vi "UHR-Fleezers Control (host) - 10.8MV_trial1.vi"() -> ()   [LabVIEW 2010] (continued)
            n273 = Concatenate Strings("1TJ3;\n2TJ3;\n3TJ3" ("Substring"), "\r") -> (w933:string)
            n274 = VISA Write(VISA resource name=w936, write buffer=w933) -> ()  [unwired: 1 in, 3 out]
          }
        }
      }
    }
  }
  n275 = disable-structure shown="Disabled" {
    disable-tunnel: w24 -> [w965 _]
    frame Disabled {
      w960 = T17 0 items=["Grayscale (U8)", "Grayscale (I16)", "Grayscale (SGL)", "Complex (CSG)", "RGB (U32)", "HSL (U32)", "RGB (U64)", "Grayscale (U16)"] ("Image Type")
      n276 = call <vilib>:"IMAQ Init.vi"("Interface Name"="img0") -> ("error out"=w962:errorcluster, "IMAQ Session Out"=w964:refnum<k11>)  [unwired: 9 in]
      n277 = call <vilib>:"IMAQ Grab Setup.vi"("error in (no error)"=w962, "IMAQ Session In"=w964) -> ("error out"=w958:errorcluster, "IMAQ Session Out"=w959:refnum<k11>)  [unwired: 8 in]
      n278 = call "IMAQ Create"("Image Name"="untitled", "Image Type"=w960) -> ("New Image"=w957:T2)  [unwired: 3 in, 1 out]
      n279 = call <vilib>:"Application Directory.vi"() -> ("Application Directory"=w944:path)
      n280 = Build Path(base path=w944, name or relative path="_trap_screen_positions") -> (appended path=w952:path)
      n281 = Open/Create/Replace File(file path (use dialog)=w952, operation (0:open)=T25."open or create", access (0:read/write)=enum16{"read/write", "read-only", "write-only"}."read/write") -> (refnum out=w954:refnum<file>)  [unwired: 3 in, 2 out]
      n282 = local read "Trap Sets"() -> (w946:u32)
      n283 = for "Load trap positions on video screen from file." {
        N: w946 -> [_]
        tunnel: [w972] -> w947
        tunnel: w954 -> [w971]
        tunnel: [w968] -> w943 mode=indexing
        w970 = 4
        n284 = for {
          N: w970 -> [_]
          tunnel: [w976] -> w972
          tunnel: w971 -> [w975]
          tunnel: w970 -> [w974]
          tunnel: [w973] -> w969 mode=indexing
          n285 = Read from Binary File(5:w974, 11:w975) -> (2:w973:i32, 3:w976:refnum<file>)  [unwired: 4 in, 2 out]
        }
        n286 = Array To Cluster(array=w969) -> (cluster=w968:T29)
      }
      n287 = node-c288() -> (w967:T26)  [unwired: 4 in]
      n288 = timed-loop "acquire video and stage position" {
        timing: w967 -> [_]
        timing-out: [_] -> w966
        tunnel: w959 -> [w995]
        tunnel: w958 -> [w994]
        tunnel: w957 -> [w993]
        tunnel: [w992] -> w939
        tunnel: [w989] -> w940
        tunnel: [w990] -> w938
        tunnel: w965 -> [_]
        shift-right: [w986] -> w956
        shift-left: w943 -> [w987]
        tunnel: w946 -> [w984]
        stop <- w991 stop-if-true
        n289 = node-c288() -> ()  [unwired: 1 in, 1 out]
        n290 = event shown="[2] \"Primary Video Display\": Mouse Down" {
          selector: _ -> [_ _ _ _]
          dyn-events: _ -> [_ _ _ _]
          timeout: 10 -> [_ _ _ _]
          tunnel: w995 -> [w1006 w1021 w1030 w1049]
          tunnel: w994 -> [w1005 w1023 w1028 w1051]
          tunnel: w993 -> [w1004 w1022 w1029 w1050]
          tunnel: [w1003 w1021 w1030 w1049] -> w992
          tunnel: [w996 w1025 FALSE FALSE] -> w991
          tunnel: [w1000 w1023 w1028 w1051] -> w990
          tunnel: [w999 w1022 w1029 w1050] -> w989
          tunnel: "radius" -> [_ _ w1035 _]
          tunnel: w987 -> [w997 w1024 w1033 _]
          tunnel: [w997 w1024 w1034 cluster{i32, i32, i32, i32}[] []] -> w986
          tunnel: w984 -> [_ _ w1026 _]
          event Timeout {
            n291 = event-data() -> ()  [unwired: 1 in, 2 out]
            n292 = call <vilib>:"IMAQ Grab Acquire.vi"("error in (no error)"=w1005, "Image In"=w1004, "IMAQ Session In"=w1006) -> ("error out"=w1001:errorcluster, "Image Out"=w1002:T2, "IMAQ Session Out"=w1003:refnum<k11>)  [unwired: 5 in, 1 out]
            n293 = case shown="True" "trap\nmarkers?" {
              tunnel: w997 -> [_ w1014]
              tunnel: w1002 -> [w1008 w1013]
              tunnel: w1001 -> [w1007 w1012]
              tunnel: [w1007 w1011] -> w1000
              tunnel: [w1008 w1009] -> w999
              frame False {
              }
              frame True {
                n294 = for {
                  tunnel: w1014 -> [w1020] mode=indexing
                  shift-right: [w1018] -> w1009
                  shift-left: w1013 -> [w1019]
                  tunnel: w1012 -> [w1017]
                  tunnel: [w1016] -> w1011
                  tunnel: u32 16711680 ("Color") -> [w1015]
                  n295 = call "IMAQ Overlay Oval"("Color"=w1015, "error in (no error)"=w1017, "Bounding Rectangle"=w1020, "Image"=w1019) -> ("error out"=w1016:errorcluster, "Image Out"=w1018:T2)  [unwired: 6 in]
                }
              }
            }
            "Primary Video Display" <- w999
            n296 = Unbundle By Name(w1001) -> ("status"=w996:bool)
          }
          event "Stop All": Value Change {
            n297 = event-data() -> ()  [unwired: 1 in, 5 out]
            n298 = local read "Stop All"() -> (w1025:bool)
          }
          event "Primary Video Display": Mouse Down {
            n299 = event-data() -> ()  [unwired: 1 in, 7 out]
            n300 = Array Size(array=w1033) -> (size(s)=w1032:i32)
            n301 = Less?(x=w1032, y=w1026) -> (x < y?=w1031:bool)
            n302 = case shown="True" w1031 {
              tunnel: w1035 -> [_ w1045]
              tunnel: w1033 -> [w1036 w1039]
              tunnel: [w1036 w1038] -> w1034
              frame False {
              }
              frame True {
                n303 = property on="Primary Video Display" class="ImageControl"() -> ("Last Mouse Position"=w1037:cluster{"X":i32, "Y":i32})  [unwired: 2 in, 2 out]
                n304 = Unbundle By Name(w1037) -> ("X"=w1047:i32, "Y"=w1046:i32)
                n305 = Add(x=w1046, y=w1045) -> (x+y=w1043:i32)
                n306 = Subtract(x=w1046, y=w1045) -> (x-y=w1041:i32)
                n307 = Add(x=w1047, y=w1045) -> (x+y=w1042:i32)
                n308 = Subtract(x=w1047, y=w1045) -> (x-y=w1044:i32)
                n309 = Bundle(w1044, w1043, w1042, w1041) -> (w1040:cluster{i32, i32, i32, i32})  [unwired: 1 in]
                n310 = Build Array (concatenate)(w1039, w1040) -> (w1038:T30)
              }
            }
          }
          event "clear markers": Value Change {
            n311 = event-data() -> ()  [unwired: 1 in, 5 out]
          }
        }
        n312 = node-c288() -> ()  [unwired: 1 in, 1 out]
      }
      n313 = node-c288(w966) -> ()  [unwired: 1 out]
      n314 = Set File Position(offset (in bytes) (0)=i64 0, refnum=w947, from (0:start)=enum16{"start", "end", "current"}."start") -> (refnum out=w948:refnum<file>)  [unwired: 1 in, 1 out]
      n315 = for "Write trap positions to file so they can be remembered\nwhen program is removed from memory" {
        tunnel: w956 -> [w980] mode=indexing
        tunnel: [w978] -> w955
        tunnel: w948 -> [w977]
        n316 = Cluster To Array(cluster=w980) -> (array=w979:i32[])
        n317 = for {
          tunnel: w979 -> [w983] mode=indexing
          tunnel: [w982] -> w978
          tunnel: w977 -> [w981]
          n318 = Write to Binary File(file (use dialog)=w981, data=w983) -> (refnum out=w982:refnum<file>)  [unwired: 4 in, 2 out]
        }
      }
      n319 = Close File(refnum=w955) -> ()  [unwired: 1 in, 2 out]
      n320 = call "IMAQ Dispose"("Image"=w940, "error in (no error)"=w938) -> ("error out"=w937:errorcluster)  [unwired: 4 in]
      n321 = call <vilib>:"IMAQ Stop.vi"("error in (no error)"=w937, "IMAQ Session In"=w939) -> ("error out"=w941:errorcluster, "IMAQ Session Out"=w942:refnum<k11>)  [unwired: 8 in]
      n322 = call <vilib>:"IMAQ Close.vi"("error in (no error)"=w941, "IMAQ Session In"=w942) -> ()  [unwired: 9 in, 1 out]
    }
    frame Enabled {
    }
  }
  n323 = node-c288(2 ("Processor")) -> (w15:T26)  [unwired: 3 in]
  n324 = node-c288() -> (w69:T26)  [unwired: 4 in]
  n325 = disable-structure shown="Enabled" {
    disable-tunnel: [w1058 _] -> w35
    disable-tunnel: w24 -> [w1057 _]
    frame Enabled {
      n326 = node-c288() -> (w1060:T26)  [unwired: 4 out]
      n327 = timed-loop "Rough control of MCL mirror stage (debugging)" {
        tunnel: w1057 -> [w1063]
        tunnel: [w1062] -> w1058
        timing: w1060 -> [_]
        timing-out: [_] -> w1059
        stop <- w1062 stop-if-true
        n328 = node-c288() -> ()  [unwired: 2 out]
        n329 = case shown="1" "MCL Mode" {
          tunnel: w1063 -> [_ w1066 w1170]
          frame 0, Default {
            # "manual positioning"
          }
          frame 1 {
            # "sinusoidal wave"
            n330 = node-c288() -> (w1068:T26)  [unwired: 4 out]
            n331 = timed-loop "Oscillate MCL mirror" {
              timing: w1068 -> [_]
              timing-out: [_] -> w1067
              tunnel: w1066 -> [w1107]
              i -> [w1106]
              stop <- w1069 stop-if-true
              n332 = node-c288() -> (w1105:i64)  [unwired: 1 out]
              n333 = Multiply(x="AO1", y=32767.0) -> (x*y=w1101:dbl)
              n334 = Multiply(x="AO2", y=32767.0) -> (x*y=w1096:dbl)
              n335 = Divide(x=w1101, y=10.0) -> (x/y=w1102:dbl)
              n336 = Divide(x=w1096, y=10.0) -> (x/y=w1097:dbl)
              n337 = To Word Integer(number=w1102) -> (16bit integer=w1094:i16)
              n338 = To Word Integer(number=w1097) -> (16bit integer=w1093:i16)
              n339 = Divide(x=w1105, y=i64 1000) -> (x/y=w1076:dbl)
              n340 = Multiply(x=w1076, y=w1106) -> (x*y=w1087:dbl)
              n341 = Multiply(x="Osc. freq. (Hz) 2", y=6.283185307179586) -> (x*y=w1088:dbl)
              n342 = Multiply(x=w1088, y=w1087) -> (x*y=w1086:dbl)
              n343 = Sine(x=w1086) -> (sin(x)=w1085:dbl)
              n344 = Multiply(x=w1085, y="Osc. amp. (V)") -> (x*y=w1083:dbl)
              n345 = Add(x=w1083, y="Osc. center (V)") -> (x+y=w1081:dbl)
              n346 = Divide(x=w1081, y=10.0) -> (x/y=w1079:dbl)
              n347 = Multiply(x=w1079, y=32767.0) -> (x*y=w1074:dbl)
              n348 = Select(t=w1074, s="Scan axis", f=w1094) -> (s? t:f=w1092:dbl)
              n349 = Select(t=w1093, s="Scan axis", f=w1074) -> (s? t:f=w1091:dbl)
              n350 = local read "MCL Mode"() -> (w1073:u16)
              n351 = Not Equal?(x=w1073, y=u16 1) -> (x != y?=w1070:bool)
              n352 = local read "Stop All"() -> (w1071:bool)
              n353 = xnode "Read/Write Control"("FPGA VI Reference In"=w1107, "AO1"=w1092, "AO2"=w1091) -> ()  [unwired: 1 in, 2 out]
              n354 = Compound Arithmetic op=OR(w1071, w1070) -> (w1069:bool)
              n355 = node-c288() -> ()  [unwired: 2 out]
            }
            n356 = node-c288(w1067) -> ()  [unwired: 1 out]
          }
          frame 2 {
            # "linear scan"
            n357 = case shown="True" "Start Scan" {
              tunnel: w1170 -> [_ w1182]
              frame False {
              }
              frame True {
                n358 = Subtract(x="End (V)", y="Begin (V)") -> (x-y=w1178:dbl)
                n359 = Decrement(x="N Points") -> (x-1=w1177:dbl)
                n360 = Divide(x=w1178, y=w1177) -> (x/y=w1175:dbl)
                n361 = for {
                  N: "N Points" -> [_]
                  tunnel: "Begin (V)" -> [w1195]
                  tunnel: w1182 -> [w1187]
                  tunnel: [w1186] -> w1181 mode=indexing
                  tunnel: w1175 -> [w1185]
                  tunnel: [w1183] -> w1174 mode=indexing
                  i -> [w1194]
                  n362 = Multiply(x=w1185, y=w1194) -> (x*y=w1193:dbl)
                  n363 = Add(x=w1195, y=w1193) -> (x+y=w1190:dbl)
                  n364 = local read "Scan axis"() -> (w1184:bool)
                  n365 = local read "AO1"() -> (w1192:dbl)
                  n366 = local read "AO2"() -> (w1191:dbl)
                  n367 = Select(t=w1190, s=w1184, f=w1192) -> (s? t:f=w1189:dbl)
                  n368 = Select(t=w1191, s=w1184, f=w1190) -> (s? t:f=w1188:dbl)
                  n369 = flat-sequence {
                    tunnel: w1189 -> [w1199]
                    tunnel: w1188 -> [w1198]
                    tunnel: w1187 -> [w1196]
                    tunnel: [w1266] -> w1186
                    tunnel: [w1265] -> w1183
                    frame #0 {
                      w1202 = 10.0 ("y")
                      w1197 = 32767.0 ("y")
                      n370 = Multiply(x=w1199, y=w1197) -> (x*y=w1205:dbl)
                      n371 = Multiply(x=w1198, y=w1197) -> (x*y=w1203:dbl)
                      n372 = Divide(x=w1205, y=w1202) -> (x/y=w1206:dbl)
                      n373 = Divide(x=w1203, y=w1202) -> (x/y=w1204:dbl)
                      n374 = To Word Integer(number=w1206) -> (16bit integer=w1200:i16)
                      n375 = To Word Integer(number=w1204) -> (16bit integer=w1201:i16)
                      n376 = xnode "Read/Write Control"("FPGA VI Reference In"=w1196, "AO1"=w1200, "AO2"=w1201) -> ()  [unwired: 1 in, 2 out]
                    }
                    frame #1 {
                      n377 = Wait (ms)(milliseconds to wait="DAQ Delay (ms)") -> ()  [unwired: 1 out]
                    }
                    frame #2 {
                      n378 = local read "Slow mean"() -> (w1266:dbl)
                      n379 = local read "Sigma"() -> (w1265:dbl)
                    }
                  }
                }
                n380 = Bundle("Begin (V)"="Begin (V)", w1175, w1181) -> (→"MCL Scan":cluster{"Begin (V)":dbl, dbl, dbl[]})  [unwired: 1 out]
                n381 = Bundle("Begin (V)"="Begin (V)", w1175, w1174) -> (→"MCL Scan 2":cluster{"Begin (V)":dbl, dbl, dbl[]})  [unwired: 1 out]
              }
            }
          }
        }
        n382 = local read "Stop All"() -> (w1062:bool)
        n383 = node-c288() -> ()  [unwired: 2 out]
      }
      n384 = node-c288(w1059) -> ()  [unwired: 1 out]
    }
    frame Disabled {
    }
  }
  n385 = timed-loop "Control parameters (event loop)" {
    tunnel: w24 -> [w1272]
    shift-right: [w1271] -> _
    shift-left: errorcluster {"status"=FALSE, "code"=0, "source"=""} ("error out") -> [w1270]
    tunnel: [w1269] -> w37
    timing: w15 -> [_]
    timing-out: [_] -> w14
    stop <- w1269 stop-if-true
    n386 = node-c288() -> ()  [unwired: 1 in, 1 out]
    n387 = event shown="[6] \"BD 1 Frequency 1 (MHz)\", \"BD 1 Frequency 2 (MHz)\", \"BD 1 Frequency 3 (MHz)\", \"BD 2 Frequency 1 (MHz)\", \"BD 2 Frequency 2 (MHz)\", \"BD 2 Frequency 3 (MHz)\", \"Trap Delta (MHz)\": Value Change" {
      selector: _ -> [_ _ _ _ _ _ _ _ _ _ _ _ _ _ _ _ _ _ _ _ _ _ _ _ _ _ _ _ _ _ _ _ _ _ _ _ _ _ _ _ _ _ _ _ _ _ _ _ _ _ _ _ _ _ _]
      dyn-events: _ -> [_ _ _ _ _ _ _ _ _ _ _ _ _ _ _ _ _ _ _ _ _ _ _ _ _ _ _ _ _ _ _ _ _ _ _ _ _ _ _ _ _ _ _ _ _ _ _ _ _ _ _ _ _ _ _]
      timeout: _ -> [_ _ _ _ _ _ _ _ _ _ _ _ _ _ _ _ _ _ _ _ _ _ _ _ _ _ _ _ _ _ _ _ _ _ _ _ _ _ _ _ _ _ _ _ _ _ _ _ _ _ _ _ _ _ _]
      tunnel: w1272 -> [w1310 _ _ _ w1432 _ w1529 _ w1593 _ _ _ w1788 _ _ w1890 w2034 w2098 w2173 w2327 w2404 w2535 w2631 w2717 w2803 w2889 w2975 w3061 w3154 w3318 w3529 _ w3674 w3811 _ w4018 w4060 w4108 w4187 w4229 _ w4275 _ _ _ _ w4466 _ w4559 w4600 w4647 w4835 w4884 _ w4946]
      tunnel: [w1309 _ _ _ w1422 _ w1528 _ w1556 _ w1753 _ w1767 _ _ w1889 w2030 w2095 w2170 w2326 w2402 w2534 w2625 w2711 w2797 w2883 w2969 w3055 w3152 w3317 w3527 _ w3672 w3809 _ w4016 w4058 w4098 w4185 w4227 _ w4273 _ _ _ _ w4464 _ _ _ _ _ _ _ _] -> w1271
      tunnel: w1270 -> [w1308 _ _ _ w1431 _ w1527 _ w1588 _ w1753 _ w1787 _ _ w1888 w2029 w2094 w2169 w2325 w2403 w2533 w2630 w2716 w2802 w2888 w2974 w3060 w3153 w3316 w3528 _ w3673 w3810 _ w4017 w4059 w4107 w4186 w4228 _ w4274 _ _ _ _ w4465 _ w4558 w4599 w4646 w4834 w4883 _ w4945]
      tunnel: [_ _ _ _ _ _ _ _ _ _ w1752 _ _ _ _ _ _ _ _ _ _ _ _ _ _ _ _ _ _ _ _ _ _ _ _ _ _ _ _ _ _ _ _ _ _ _ _ _ _ _ _ _ _ _ _] -> w1269
      tunnel: [_ _ _ _ _ _ _ "Round T1 X" _ _ _ _ _ _ _ _ _ _ _ _ _ _ _ _ _ _ _ _ _ _ _ _ _ _ _ _ _ _ _ _ _ _ _ _ _ _ _ _ _ _ _ _ _ _ _] -> _
      tunnel: [_ _ _ "Adjust Scale\nto Mean" _ _ _ _ _ _ _ _ _ _ _ _ _ _ _ _ _ _ _ _ _ _ _ _ _ _ _ _ _ _ _ _ _ _ _ _ _ _ _ _ _ _ _ _ _ _ _ _ "Set SP to Reading" _ _] -> _
      tunnel: [_ _ _ _ _ _ _ _ _ "Round T2 X" _ "Delayed Interlace Start" _ _ _ _ _ _ _ _ _ _ _ _ _ _ _ _ _ _ _ _ _ _ _ _ _ _ _ _ _ _ _ _ _ _ _ _ _ _ _ _ _ _ _] -> _
      event "AI Count (ticks)", "Sets to FIFO (Traps)", "Save ave N", "FPGA Ave.", "# Samples/channel", "N sets to save": Value Change {
        # "So that if 'Save ave N' is updated, the AOD scanning code updates too."
        n388 = event-data() -> ()  [unwired: 6 out]
        n389 = local read "AI Count (ticks)"() -> (w1290:u32)
        n390 = Boolean To (0,1)(Boolean="Sets to FIFO (Traps)") -> (0, 1=w1300:cluster{"Set 1":i16, "Set 2":i16, "Set 3":i16})
        n391 = xnode "Read/Write Control"("FPGA VI Reference In"=w1310, "error in"=w1308, "ai count"=w1290, "AI1 Sets to FIFO"="Sets to FIFO (Traps)", "N of AI1 Int Acq Sets"="N Acq Sets (Traps + Fl.)") -> ("error out"=w1309:errorcluster)  [unwired: 1 out]
        n392 = Cluster To Array(cluster=w1300) -> (array=w1299:i16[])
        n393 = To Unsigned Long Integer(number=w1299) -> (unsigned 32bit integer=w1279:u32[])
        n394 = local read "Scan steps (AOD)"() -> (w1301:u64)
        n395 = Multiply(x=w1290, y="N Acq Sets (Traps + Fl.)") -> (x*y=w1288:u32)
        n396 = Divide(x=40000000.0, y=w1290) -> (x/y=w1282:dbl)
        "AI rate (Hz)" <- w1282
        "Ave. Rate (Hz)" <- w1282
        n397 = Add Array Elements(numeric array=w1279) -> (sum=w1291:u32)
        "Trap Sets" <- w1291
        n398 = Reciprocal(x=w1282) -> (1/x=→"Ave. Period (s)":dbl)
        n399 = property on="Scan steps (AOD)" class="DigNum (strict)"("Val(Sgnl)"=w1301) -> ()  [unwired: 2 in, 2 out]
        n400 = Divide(x=w1282, y="N Acq Sets (Traps + Fl.)") -> (x/y=w1305:dbl)
        "Data Rate (Hz)" <- w1305
        n401 = Reciprocal(x=w1305) -> (1/x=→"Data Period (s)":dbl)
        n402 = local read "Save ave N"() -> (w1304:dbl)
        n403 = Divide(x=w1305, y=w1304) -> (x/y=w1303:dbl)
        "Save Data Rate (Hz)" <- w1303
        n404 = Reciprocal(x=w1303) -> (1/x=→"Save Data Period (s)":dbl)
        n405 = Multiply(x=w1288, y="# Samples/trap") -> (x*y=w1286:u32)
        "Counts/DMA" <- w1286
        n406 = property on="Trap Disp. Downsample" class="DigNum (strict)"("Maximum"="# Samples/trap") -> ()  [unwired: 2 in, 2 out]
        n407 = Multiply(x=w1291, y="# Samples/trap") -> (x*y=w1280:u32)
        "# Samples/channel" <- w1280
        n408 = Multiply(x=w1280, y=u32 8) -> (x*y=→"Trap AI Elements/DMA read":u32)
        n409 = local read "APD Int. Count"() -> (w1287:u32)
        n410 = Multiply(x=w1280, y=u32 3) -> (x*y=→"Trap Pos Elements/DMA read":u32)
        n411 = Divide(x=w1286, y=w1287) -> (x/y=w1277:dbl)
        "APD Samples/FIFO Acq." <- w1277
        n412 = Divide(x=w1286, y=40000000.0) -> (x/y=w1284:dbl)
        "DMA Update Period (s)" <- w1284
        n413 = Multiply(x=2.0, y=w1277) -> (x*y=→"APD Elements/DMA read":dbl)
        n414 = property on="APD Disp. Downsample" class="DigNum (strict)"("Maximum"=w1277) -> ()  [unwired: 2 in, 2 out]
        n415 = local read "N sets to save"() -> (w1297:u32)
        n416 = Multiply(x=w1284, y=w1297) -> (x*y=→"Total Time (s)":dbl)
        "FPGA Averaging" <- FALSE ("FPGA Averaging")
      }
      event "Rescale on Mean": Value Change {
        n417 = event-data() -> ()  [unwired: 7 out]
        n418 = And(x=FALSE, y="Rescale on Mean") -> (x .and. y?=w1397:bool)
        n419 = local write "Rescale on Mean"(w1397) -> ()
        n420 = local read "Bead Mean (nm)"() -> (w1402:dbl)
        n421 = Add(x="Amplitude (nm)", y=w1402) -> (x+y=w1400:dbl)
        n422 = Subtract(x=w1402, y="Amplitude (nm)") -> (x-y=w1399:dbl)
        n423 = property on="Bead Separation" class="WFChart (strict)"("YScale.Minimum"=w1399) -> ()  [unwired: 2 in, 2 out]
        n424 = property on="Bead Separation" class="WFChart (strict)"("YScale.Maximum"=w1400) -> ()  [unwired: 2 in, 2 out]
      }
      event "Detector Type": Value Change {
        n425 = event-data() -> ()  [unwired: 7 out]
        n426 = local read "AI labels"() -> (w1403:string[])
        n427 = property on="High Res. Display" class="Ring (strict)"("Strings []"=w1403) -> ()  [unwired: 2 in, 2 out]
        n428 = Build Array (concatenate)(w1403, "none") -> (w1404:string[])
        n429 = property on="FFT 1 Choice 1" class="Ring (strict)"("Strings []"=w1404) -> ()  [unwired: 2 in, 2 out]
        n430 = property on="FFT 1 Choice 2" class="Ring (strict)"("Strings []"=w1404) -> ()  [unwired: 2 in, 2 out]
        n431 = property on="FFT 2 Choice 1" class="Ring (strict)"("Strings []"=w1404) -> ()  [unwired: 2 in, 2 out]
        n432 = property on="FFT 2 Choice 2" class="Ring (strict)"("Strings []"=w1404) -> ()  [unwired: 2 in, 2 out]
        n433 = Bundle("APD 1", "APD 2") -> (w1407:cluster{string, string})  [unwired: 1 out]
        n434 = Cluster To Array(cluster=w1407) -> (array=w1405:string[])
        n435 = Build Array (concatenate)(w1405, w1404) -> (w1409:string[])
        n436 = Array Size(array=w1409) -> (size(s)=w1410:i32)
        n437 = property on="Signals to Plot" class="LstBox (strict)"("Item Names"=w1409) -> ()  [unwired: 2 in, 2 out]
        n438 = property on="Signals to Plot" class="LstBox (strict)"("Number of Rows"=w1410) -> ()  [unwired: 2 in, 2 out]
        n439 = property on="All Signals" class="WFChart (strict)"("LegNumRows"=w1410) -> ()  [unwired: 2 in, 2 out]
      }
      event "Adjust Scale\nto Mean": Value Change {
        n440 = event-data() -> ()  [unwired: 7 out]
        n441 = local read "APD 1 Rate (Hz)"() -> (w1419:dbl)
        n442 = Multiply(x=1000.0, y="Above (kHz)") -> (x*y=w1417:dbl)
        n443 = Multiply(x=1000.0, y="Below (kHz)") -> (x*y=w1415:dbl)
        n444 = Add(x=w1417, y=w1419) -> (x+y=w1412:dbl)
        n445 = Subtract(x=w1419, y=w1415) -> (x-y=w1413:dbl)
        n446 = property on="APD Chart" class="WFChart (strict)"("YScale.Minimum"=w1413) -> ()  [unwired: 2 in, 2 out]
        n447 = property on="APD Chart" class="WFChart (strict)"("YScale.Maximum"=w1412) -> ()  [unwired: 2 in, 2 out]
      }
      event "Phase adj. (AI1)", "+ phase (AI1)", "- phase (AI1)": Value Change {
        n448 = event-data() -> ()  [unwired: 7 out]
        n449 = Negate(x="Phase adj. (AI1)") -> (-x=w1429:i16)
        n450 = Select(t=w1429, s="- phase (AI1)", f="Phase adj. (AI1)") -> (s? t:f=w1428:i16)
        n451 = xnode "Read/Write Control"("FPGA VI Reference In"=w1432, "error in"=w1431, "Phase count adjustment"=w1428) -> ("FPGA VI Reference Out"=w1427:T19, "error out"=w1426:errorcluster)
        n452 = Or(x="- phase (AI1)", y="+ phase (AI1)") -> (x .or. y?=w1423:bool)
        n453 = xnode "Read/Write Control"("FPGA VI Reference In"=w1427, "error in"=w1426, "+ phase"=w1423) -> ("error out"=w1422:errorcluster)  [unwired: 1 out]
      }
      event "Signals to Plot": Double Click {
        w1510 = u32 9868950 ("Color Box")
        n454 = event-data() -> ("Row"=w1512:i32)  [unwired: 9 out]
        n455 = property on="All Signals" class="WFChart (strict)"("Active Plot"=w1512) -> (error out=w1523:errorcluster)  [unwired: 2 in, 1 out]
        n456 = property on="All Signals" class="WFChart (strict)" props=["Plot", "Visible?", "Plot", "Plot Color"](error in=w1523) -> (error out=w1522:errorcluster, "Plot.Visible?"=w1521:bool)  [unwired: 1 in, 2 out]
        n457 = Select(t=FALSE ("Plot.Visible"), s=w1521, f=TRUE ("Plot.Visible")) -> (s? t:f=w1516:bool)
        n458 = property on="All Signals" class="WFChart (strict)"(error in=w1522, "Plot.Visible?"=w1516) -> (error out=w1518:errorcluster)  [unwired: 1 in, 1 out]
        n459 = property on="All Signals" class="WFChart (strict)"(error in=w1518) -> (error out=w1513:errorcluster, "Plot.Plot Color"=w1517:u32)  [unwired: 1 in, 1 out]
        n460 = property on="Signals to Plot" class="LstBox (strict)"(error in=w1513, "Active Row"=w1512) -> (error out=w1511:errorcluster)  [unwired: 1 in, 1 out]
        n461 = Select(t=w1517, s=w1516, f=u32 0) -> (s? t:f=w1514:u32)
        n462 = property on="Signals to Plot" class="LstBox (strict)"(error in=w1511, "CellFontColor"=w1514, "SelColor"=w1510, "CellBG"=w1510, "CellFontSize"=u32 20 ("Active Row:Cell Font:Size"), "CellFontBold"=TRUE ("Active Row:Cell Font:Bold")) -> ()  [unwired: 1 in, 2 out]
      }
      event "BD 1 Frequency 1 (MHz)", "BD 1 Frequency 2 (MHz)", "BD 1 Frequency 3 (MHz)", "BD 2 Frequency 1 (MHz)", "BD 2 Frequency 2 (MHz)", "BD 2 Frequency 3 (MHz)", "Trap Delta (MHz)": Value Change {
        # "anytime one of the frequencies is changed, write it to the RF board UNLESS Set 2 is being oscillated. The oscillation\nscript writes the frequencies to the RF board."
        n463 = event-data() -> ("CtlRef"=w1526:refnum<vi>)  [unwired: 6 out]
        n464 = control-ref of="Trap Delta (MHz)"() -> (w1525:refnum<vi>)
        n465 = Equal?(x=w1525, y=w1526) -> (x = y?=w1524:bool)
        n466 = case shown="False" "Oscillate Set 2" {
          tunnel: w1529 -> [w1549 _]
          tunnel: [w1548 w1552] -> w1528
          tunnel: w1527 -> [w1547 w1552]
          tunnel: w1524 -> [w1533 _]
          frame False {
            n467 = local read "BD 1 Frequency 1 (MHz)"() -> (w1531:dbl)
            n468 = local read "BD 1 Frequency 2 (MHz)"() -> (w1535:dbl)
            n469 = Add(x=w1531, y="Trap Delta (MHz)") -> (x+y=w1534:dbl)
            n470 = Select(t=w1534, s=w1533, f=w1535) -> (s? t:f=w1532:dbl)
            n471 = local read "Y RF Frequency Limits (MHz)"() -> (w1537:T16)
            n472 = local read "X RF Frequency Limits (MHz)"() -> (w1538:T16)
            n473 = local read "BD 1 Frequency 3 (MHz)"() -> (w1550:dbl)
            n474 = local write "BD 1 Frequency 2 (MHz)"(w1532) -> ()
            n475 = local read "BD 2 Frequency 1 (MHz)"() -> (w1541:dbl)
            n476 = local read "BD 2 Frequency 2 (MHz)"() -> (w1540:dbl)
            n477 = local read "BD 2 Frequency 3 (MHz)"() -> (w1551:dbl)
            n478 = call "set RF board frequency - interlace.vi"("Board 2 Frequency Limits"=w1537, "Board 1 Frequency Limits"=w1538, "error in"=w1547, "FPGA VI Reference In"=w1549, "Board 2 Frequency 3 (MHz)"=w1551, "Board 1 Frequency 3 (MHz)"=w1550, "Board 2 Frequency 2 (MHz)"=w1540, "Board 2 Frequency 1 (MHz)"=w1541, "Board 1 Frequency 2 (MHz)"=w1532, "Board 1 Frequency 1  (MHz)"=w1531) -> ("error out"=w1548:errorcluster)  [unwired: 1 out]
            n479 = Subtract(x=w1541, y=w1540) -> (x-y=w1545:dbl)
            n480 = Subtract(x=w1532, y=w1531) -> (x-y=w1546:dbl)
            n481 = Square(x=w1545) -> (x^2=w1543:dbl)
            n482 = Square(x=w1546) -> (x^2=w1544:dbl)
            n483 = Add(x=w1544, y=w1543) -> (x+y=w1542:dbl)
            n484 = Square Root(x=w1542) -> (sqrt(x)=w1539:dbl)
            n485 = local write "Trap Delta (MHz)"(w1539) -> ()
            n486 = property on="Initial delta (MHz)" class="DigNum (strict)"("Val(Sgnl)"=w1539) -> ()  [unwired: 2 in, 2 out]
          }
          frame True {
          }
        }
      }
      event "Round T1 X": Value Change {
        n487 = event-data() -> ()  [unwired: 7 out]
        n488 = local read "BD 1 Frequency 1 (MHz)"() -> (w1555:dbl)
        n489 = Round To Nearest(number=w1555) -> (nearest integer value=w1554:dbl)
        n490 = property on="BD 1 Frequency 1 (MHz)" class="DigNum (strict)"("Val(Sgnl)"=w1554) -> ()  [unwired: 2 in, 2 out]
      }
      event "Restart RF": Value Change {
        n491 = event-data() -> ()  [unwired: 7 out]
        n492 = xnode "Read/Write Control"("FPGA VI Reference In"=w1593, "error in"=w1588, "FPGA Controls  RF Box"=FALSE) -> ("FPGA VI Reference Out"=w1592:T19, "error out"=w1587:errorcluster)
        n493 = local read "Y RF Amplitude Limits (%)"() -> (w1568:T16)
        n494 = local read "X RF Amplitude Limits (%)"() -> (w1569:T16)
        n495 = local read "X RF Frequency Limits (MHz)"() -> (w1571:T16)
        n496 = local read "Y RF Frequency Limits (MHz)"() -> (w1570:T16)
        n497 = xnode "Read/Write Control"("FPGA VI Reference In"=w1592, "error in"=w1587, "Direct RF Box  Communication"=TRUE) -> ("FPGA VI Reference Out"=w1591:T19, "error out"=w1586:errorcluster)
        n498 = local read "BD 2 Frequency 3 (MHz)"() -> (w1578:dbl)
        n499 = local read "BD 2 Frequency 2 (MHz)"() -> (w1579:dbl)
        n500 = local read "BD 1 Frequency 3 (MHz)"() -> (w1582:dbl)
        n501 = local read "BD 1 Frequency 1 (MHz)"() -> (w1583:dbl)
        n502 = local read "BD 2 Frequency 1 (MHz)"() -> (w1580:dbl)
        n503 = local read "BD 1 Frequency 2 (MHz)"() -> (w1581:dbl)
        n504 = call "Initialize RF boards - interlace 3.vi"("error in"=w1586, "FPGA VI Reference In"=w1591) -> ("error out"=w1585:errorcluster, "FPGA VI Reference Out"=w1590:T19)
        n505 = local read "BD 2 Amplitude 2 (%)"() -> (w1573:dbl)
        n506 = local read "BD 2 Amplitude 1 (%)"() -> (w1574:dbl)
        n507 = local read "BD 2 Amplitude 3 (%)"() -> (w1572:dbl)
        n508 = local read "BD 1 Amplitude 3 (%)"() -> (w1577:dbl)
        n509 = local read "BD 1 Amplitude 1 (%)"() -> (w1576:dbl)
        n510 = local read "BD 1 Amplitude 2 (%)"() -> (w1575:dbl)
        n511 = call "set RF board frequency - interlace.vi"("Board 2 Frequency Limits"=w1570, "Board 1 Frequency Limits"=w1571, "error in"=w1585, "FPGA VI Reference In"=w1590, "Board 2 Frequency 3 (MHz)"=w1578, "Board 1 Frequency 3 (MHz)"=w1582, "Board 2 Frequency 2 (MHz)"=w1579, "Board 2 Frequency 1 (MHz)"=w1580, "Board 1 Frequency 2 (MHz)"=w1581, "Board 1 Frequency 1  (MHz)"=w1583) -> ("error out"=w1584:errorcluster, "FPGA VI Reference Out"=w1589:T19)
        n512 = call "set RF board amplitude - interlace.vi"("Board 2 Amplitude Limits"=w1568, "Board 1 Amplitude Limits"=w1569, "error in"=w1584, "FPGA VI Reference In"=w1589, "Board 2 Amplitude 3 (%)"=w1572, "Board 1 Amplitude 3 (%)"=w1577, "Board 2 Amplitude 2 (%)"=w1573, "Board 2 Amplitude 1 (%)"=w1574, "Board 1 Amplitude 2 (%)"=w1575, "Board 1 Amplitude 1 (%)"=w1576) -> ("error out"=w1561:errorcluster, "FPGA VI Reference Out"=w1565:T19)
        n513 = xnode "Read/Write Control"("FPGA VI Reference In"=w1565, "error in"=w1561, "Direct RF Box  Communication"=FALSE) -> ("FPGA VI Reference Out"=w1564:T19, "error out"=w1563:errorcluster)
        n514 = flat-sequence {
          tunnel: w1563 -> [w1594]
          tunnel: [w1594] -> w1562
          frame #0 {
            n515 = Wait (ms)(milliseconds to wait=u32 50) -> ()  [unwired: 1 out]
          }
        }
        n516 = xnode "Read/Write Control"("FPGA VI Reference In"=w1564, "error in"=w1562, "FPGA Controls  RF Box"=TRUE) -> ("error out"=w1557:errorcluster)  [unwired: 1 out]
        n517 = property on="Restart RF" class="Bool (strict)"(error in=w1557, "Value"=FALSE ("Restart RF")) -> (error out=w1556:errorcluster)  [unwired: 1 in, 1 out]
      }
      event "Round T2 X": Value Change {
        n518 = event-data() -> ()  [unwired: 7 out]
        n519 = local read "BD 1 Frequency 2 (MHz)"() -> (w1749:dbl)
        n520 = Round To Nearest(number=w1749) -> (nearest integer value=w1748:dbl)
        n521 = property on="BD 1 Frequency 2 (MHz)" class="DigNum (strict)"("Val(Sgnl)"=w1748) -> ()  [unwired: 2 in, 2 out]
      }
      event "Stop All": Value Change {
        n522 = event-data() -> ()  [unwired: 7 out]
        n523 = call "hamilton_controller.vi"("action"=T22."DISCONNECT") -> ()  [unwired: 10 in, 1 out]
        n524 = local read "Stop All"() -> (w1752:bool)
      }
      event "Delayed Interlace Start": Value Change {
        n525 = event-data() -> ()  [unwired: 7 out]
        n526 = flat-sequence {
          frame #0 {
            n527 = Multiply(x="Delay to Interlace (s)", y=1000.0) -> (x*y=w1755:dbl)
            n528 = Wait (ms)(milliseconds to wait=w1755) -> ()  [unwired: 1 out]
          }
          frame #1 {
            n529 = property on="Green laser mode" class="RadioBtnsControl (strict)"("Val(Sgnl)"=enum32{"Laser ON", "Laser OFF", "Interlace"}."Interlace" ("Value (Signaling)")) -> ()  [unwired: 2 in, 2 out]
          }
        }
      }
      event "BD 1 Amplitude 1 (%)", "BD 1 Amplitude 2 (%)", "BD 1 Amplitude 3 (%)", "BD 2 Amplitude 1 (%)", "BD 2 Amplitude 2 (%)", "BD 2 Amplitude 3 (%)", "Trap 1 ON", "Trap 2 ON", "Trap 3 ON", "Feedback On/Off", "All FB On/Off": Value Change {
        w1779 = i16 1 ("f")
        n530 = event-data() -> ()  [unwired: 7 out]
        n531 = local write "Trap 1 (ON/OFF)"("Trap 1 ON") -> ()
        n532 = local write "Trap 2 (ON/OFF)"("Trap 2 ON") -> ()
        n533 = Boolean To (0,1)(Boolean="Trap 3 ON") -> (0, 1=w1780:i16)
        n534 = Boolean To (0,1)(Boolean="Trap 1 ON") -> (0, 1=w1781:i16)
        n535 = Boolean To (0,1)(Boolean="Trap 2 ON") -> (0, 1=w1782:i16)
        n536 = Select(t=w1782, s="Trap ON/OFF X or Y Amp?", f=w1779) -> (s? t:f=w1777:i16)
        n537 = Select(t=w1781, s="Trap ON/OFF X or Y Amp?", f=w1779) -> (s? t:f=w1778:i16)
        n538 = Select(t=w1780, s="Trap ON/OFF X or Y Amp?", f=w1779) -> (s? t:f=w1776:i16)
        n539 = Select(t=w1779, s="Trap ON/OFF X or Y Amp?", f=w1782) -> (s? t:f=w1774:i16)
        n540 = Select(t=w1779, s="Trap ON/OFF X or Y Amp?", f=w1781) -> (s? t:f=w1775:i16)
        n541 = Select(t=w1779, s="Trap ON/OFF X or Y Amp?", f=w1780) -> (s? t:f=w1773:i16)
        n542 = And(x="All FB On/Off", y="Feedback On/Off") -> (x .and. y?=w1771:cluster{"Set 1":bool, "Set 2":bool})
        n543 = local read "BD 1 Amplitude 1 (%)"() -> (w1791:dbl)
        n544 = local read "BD 1 Amplitude 2 (%)"() -> (w1790:dbl)
        n545 = local read "BD 1 Amplitude 3 (%)"() -> (w1789:dbl)
        n546 = Unbundle By Name(w1771) -> ("Set 1"=w1766:bool, "Set 2"=w1763:bool)
        n547 = local read "Y RF Amplitude Limits (%)"() -> (w1759:T16)
        n548 = local read "X RF Amplitude Limits (%)"() -> (w1760:T16)
        n549 = local read "BD 2 Amplitude 1 (%)"() -> (w1792:dbl)
        n550 = local read "BD 2 Amplitude 2 (%)"() -> (w1793:dbl)
        n551 = local read "BD 2 Amplitude 3 (%)"() -> (w1794:dbl)
        n552 = And(x="Trap 2 ON", y=w1763) -> (x .and. y?=w1761:bool)
        n553 = And(x="Trap 1 ON", y=w1766) -> (x .and. y?=w1764:bool)
        n554 = Multiply(x=w1778, y=w1791) -> (x*y=w1786:dbl)
        n555 = Multiply(x=w1790, y=w1777) -> (x*y=w1784:dbl)
        n556 = Multiply(x=w1789, y=w1776) -> (x*y=w1785:dbl)
        n557 = Multiply(x=w1792, y=w1775) -> (x*y=w1795:dbl)
        n558 = Multiply(x=w1793, y=w1774) -> (x*y=w1796:dbl)
        n559 = Multiply(x=w1794, y=w1773) -> (x*y=w1797:dbl)
        n560 = call "set RF board amplitude - interlace.vi"("Board 2 Amplitude Limits"=w1759, "Board 1 Amplitude Limits"=w1760, "error in"=w1787, "FPGA VI Reference In"=w1788, "Board 2 Amplitude 3 (%)"=w1797, "Board 1 Amplitude 3 (%)"=w1785, "Board 2 Amplitude 2 (%)"=w1796, "Board 2 Amplitude 1 (%)"=w1795, "Board 1 Amplitude 2 (%)"=w1784, "Board 1 Amplitude 1 (%)"=w1786) -> ("error out"=w1768:errorcluster, "FPGA VI Reference Out"=w1769:T19)
        n561 = xnode "Read/Write Control"("FPGA VI Reference In"=w1769, "error in"=w1768, "FB On/Off Set 1"=w1764, "FB On/Off Set 2"=w1761) -> ("error out"=w1767:errorcluster)  [unwired: 1 out]
      }
      event "Load parameters": Value Change {
        n562 = event-data() -> ()  [unwired: 7 out]
        n563 = property on="Saved AOD Raster Scan Parameter Sets" class="Arr (strict)"() -> ("Index Values"=w1867:u32[])  [unwired: 2 in, 2 out]
        n564 = Index Array(array=w1867, index=0) -> (element=w1864:u32)
        n565 = local write "Load parameters"(FALSE ("Load parameters")) -> ()
        n566 = Index Array(array="Saved AOD Raster Scan Parameter Sets", index=w1864) -> (element=w1863:T32)
        n567 = Unbundle By Name(w1863) -> ("Scan Range AOD (nm) 2"=w1862:dbl, "Step Size AOD (nm) 2"=w1861:dbl, "Scan Speed AOD (nm/s) 2"=w1860:dbl, "Number of scans (AOD) 2"=w1859:u16)
        n568 = flat-sequence {
          tunnel: w1862 -> [w1870]
          tunnel: w1861 -> [w1869]
          tunnel: w1860 -> [w1868]
          tunnel: w1859 -> [w1871]
          frame #0 {
            n569 = local write "Scan Speed (nm/s)"(w1868) -> ()
            n570 = local write "Scan Range (nm)"(w1870) -> ()
            n571 = local write "Step Size (nm)"(w1869) -> ()
          }
          frame #1 {
            n572 = property on="Number of F/B Scans (AOD)" class="DigNum (strict)"("Val(Sgnl)"=w1871) -> ()  [unwired: 2 in, 2 out]
          }
        }
      }
      event "Trap 1 (ON/OFF)", "Trap 2 (ON/OFF)": Value Change {
        n573 = event-data() -> ()  [unwired: 7 out]
        n574 = property on="Trap 2 ON" class="Bool (strict)"("Val(Sgnl)"="Trap 2 (ON/OFF)") -> ()  [unwired: 2 in, 2 out]
        n575 = property on="Trap 1 ON" class="Bool (strict)"("Val(Sgnl)"="Trap 1 (ON/OFF)") -> ()  [unwired: 2 in, 2 out]
      }
      event "DIO count 1 (ticks)", "DIO count 2 (ticks)", "DIO count 3 (ticks)", "Interlace", "Number Interlace Sets", "Not-Interlacing Set": Value Change {
        n576 = event-data() -> ()  [unwired: 7 out]
        n577 = local read "DIO count 3 (ticks)"() -> (w1884:u32)
        n578 = local read "DIO count 1 (ticks)"() -> (w1886:u32)
        n579 = local read "DIO count 2 (ticks)"() -> (w1885:u32)
        n580 = To Unsigned Byte Integer(number="Not-Interlacing Set") -> (unsigned 8bit integer=w1875:u8)
        n581 = Add(x=w1875, y=u8 1) -> (x+y=w1879:u8)
        n582 = xnode "Read/Write Control"("FPGA VI Reference In"=w1890, "error in"=w1888, "DIO count 1 (ticks)"=w1886, "DIO count 2 (ticks)"=w1885, "DIO count 3 (ticks)"=w1884, "Interlace ON/OFF"="Interlace", "Number Interlace Cycles"="Number Interlace Sets", "Interlace Off Parameters"=w1879) -> ("error out"=w1889:errorcluster)  [unwired: 1 out]
        n583 = Build Array(w1886, w1885, w1884) -> (w1877:u32[])
        n584 = Split 1D Array(array=w1877, index="Number Interlace Sets") -> (first subarray=w1887:u32[])  [unwired: 1 out]
        n585 = Index Array(array=w1877, index=w1875) -> (element=w1876:u32)
        n586 = Add Array Elements(numeric array=w1887) -> (sum=w1881:u32)
        n587 = Select(t=w1881, s="Interlace", f=w1876) -> (s? t:f=→"Total Counts (ticks)":u32)
      }
      event "Reset Feedback": Value Change {
        n588 = event-data() -> ()  [unwired: 7 out]
        n589 = Unbundle By Name("Reset Feedback") -> ("Set 1"=w2032:bool, "Set 2"=w2031:bool)
        n590 = xnode "Read/Write Control"("FPGA VI Reference In"=w2034, "error in"=w2029, "FB Reset Set 1"=w2032, "FB Reset Set 2"=w2031) -> ("error out"=w2030:errorcluster)  [unwired: 1 out]
      }
      event "PID Gains": Value Change {
        n591 = event-data() -> ()  [unwired: 7 out]
        n592 = Unbundle By Name("PID Gains") -> ("Set 1"=w2097:T14, "Set 2"=w2096:T14)
        n593 = xnode "Read/Write Control"("FPGA VI Reference In"=w2098, "error in"=w2094, "FB Gains Set 1"=w2097, "FB Gains Set 2"=w2096) -> ("error out"=w2095:errorcluster)  [unwired: 1 out]
      }
      event "AI2 to Setpoint", "Trap Intensity\nSetpoints (V)": Value Change {
        n594 = event-data() -> ()  [unwired: 7 out]
        n595 = xnode "Read/Write Control"("FPGA VI Reference In"=w2173, "error in"=w2169) -> ("FPGA VI Reference Out"=w2172:T19, "error out"=w2171:errorcluster, "AI2 Y Sum Set 1"=w2180:i16, "AI2 Y Sum Set 2"=w2179:i16)
        n596 = Cluster To Array(cluster="AI2 to Setpoint") -> (array=w2183:bool[])
        n597 = local read "AI2 (V)"() -> (w2181:cluster{"Set 1":dbl, "Set 2":dbl})
        n598 = Or Array Elements(Boolean array=w2183) -> (logical OR=w2184:bool)
        n599 = Bundle By Name(cluster=w2181, "Set 1"=w2180, "Set 2"=w2179) -> (w2178:cluster{"Set 1":dbl, "Set 2":dbl})
        n600 = Divide(x=w2178, y=3276.7) -> (x/y=w2177:cluster{"Set 1":dbl, "Set 2":dbl})
        "AI2 (V)" <- w2177
        n601 = case shown="True" w2184 {
          tunnel: [w2248 w2265] -> w2176
          tunnel: "AI2 to Setpoint" -> [_ w2261]
          tunnel: "Trap Intensity\nSetpoints (V)" -> [w2249 w2264]
          tunnel: w2177 -> [_ w2258]
          frame False {
            n602 = Multiply(x=3276.7, y=w2249) -> (x*y=w2250:cluster{"Set 1":dbl, "Set 2":dbl})
            n603 = To Word Integer(number=w2250) -> (16bit integer=w2248:cluster{"Set 1":i16, "Set 2":i16})
          }
          frame True {
            n604 = Unbundle By Name(w2258) -> ("Set 1"=w2257:dbl, "Set 2"=w2256:dbl)
            n605 = Unbundle By Name(w2264) -> ("Set 1"=w2263:dbl, "Set 2"=w2262:dbl)
            n606 = Unbundle By Name(w2261) -> ("Set 1"=w2260:bool, "Set 2"=w2259:bool)
            n607 = Select(t=w2257, s=w2260, f=w2263) -> (s? t:f=w2255:dbl)
            n608 = Select(t=w2256, s=w2259, f=w2262) -> (s? t:f=w2254:dbl)
            n609 = Bundle By Name(cluster=w2264, "Set 1"=w2255, "Set 2"=w2254) -> (w2252:cluster{"Set 1":dbl, "Set 2":dbl})
            n610 = local write "Trap Intensity\nSetpoints (V)"(w2252) -> ()
            n611 = Multiply(x=3276.7, y=w2252) -> (x*y=w2253:cluster{"Set 1":dbl, "Set 2":dbl})
            n612 = To Word Integer(number=w2253) -> (16bit integer=w2265:cluster{"Set 1":i16, "Set 2":i16})
          }
        }
        n613 = Unbundle By Name(w2176) -> ("Set 1"=w2175:i16, "Set 2"=w2174:i16)
        n614 = xnode "Read/Write Control"("FPGA VI Reference In"=w2172, "error in"=w2171, "FB Setpoint Set 1"=w2175, "FB Setpoint Set 2"=w2174) -> ("error out"=w2170:errorcluster)  [unwired: 1 out]
      }
      event "Invert GI": Value Change {
        n615 = event-data() -> ()  [unwired: 7 out]
        n616 = xnode "Read/Write Control"("FPGA VI Reference In"=w2327, "error in"=w2325, "Invert GI"="Invert GI", "Invert GI 2"="Invert GI") -> ("error out"=w2326:errorcluster)  [unwired: 1 out]
      }
      event "Green FB Setpoint (mV)", "Green FB Gains", "Green FB On/Off", "Current When FB OFF (%)", "Green int current ON count adj": Value Change {
        n617 = event-data() -> ()  [unwired: 7 out]
        n618 = local read "Green FB Setpoint (mV)"() -> (w2393:dbl)
        n619 = local read "Current When FB OFF (%)"() -> (w2396:dbl)
        n620 = Multiply(x=w2393, y=3.2767) -> (x*y=w2392:dbl)
        n621 = Multiply(x=w2396, y=655.35) -> (x*y=w2397:dbl)
        n622 = To Unsigned Word Integer(number=w2397) -> (unsigned 16bit integer=w2395:u16)
        n623 = local read "Green int current ON count adj"() -> (w2400:u32)
        n624 = local read "Green FB Gains"() -> (w2399:T14)
        n625 = local read "Green Laser ON/Interlacing"() -> (w2390:bool)
        n626 = local read "Green laser mode"() -> (w2389:enum32{"Laser ON", "Laser OFF", "Interlace"})
        n627 = local read "Green FB On/Off"() -> (w2401:bool)
        n628 = Equal?(x=w2389, y=enum32{"Laser ON", "Laser OFF", "Interlace"}."Interlace") -> (x = y?=w2387:bool)
        n629 = Compound Arithmetic op=AND(w2387, w2401, w2390) -> (w2391:bool)
        n630 = xnode "Read/Write Control"("FPGA VI Reference In"=w2404, "error in"=w2403, "Green FB Setpoint"=w2392, "Green FB On/Off"=w2391, "Current Out"=w2395, "Green int current ON count adj"=w2400, "Green FB Gains"=w2399) -> ("error out"=w2402:errorcluster)  [unwired: 1 out]
      }
      event "Green laser mode", "Green Laser ON/Interlacing": Value Change {
        n631 = event-data() -> ()  [unwired: 7 out]
        n632 = case shown="True" "Green Laser ON/Interlacing" {
          tunnel: "Green laser mode" -> [_ w2542]
          tunnel: [enum32{"Laser ON", "Laser OFF", "Interlace"}."Laser OFF" ("Green laser mode") w2542] -> w2530
          tunnel: [FALSE w2538] -> w2529
          frame False {
          }
          frame True {
            n633 = local read "Green FB On/Off"() -> (w2539:bool)
            n634 = Equal?(x=w2542, y=enum32{"Laser ON", "Laser OFF", "Interlace"}."Interlace") -> (x = y?=w2540:bool)
            n635 = And(x=w2540, y=w2539) -> (x .and. y?=w2538:bool)
          }
        }
        n636 = xnode "Read/Write Control"("FPGA VI Reference In"=w2535, "error in"=w2533, "Operating Mode"=w2530, "Operating Mode 2"=w2530, "Green FB On/Off"=w2529) -> ("error out"=w2534:errorcluster)  [unwired: 1 out]
      }
      event "- phase (APD 1 Gate)", "+ phase (APD 1 Gate)": Value Change {
        n637 = event-data() -> ()  [unwired: 7 out]
        n638 = local read "Phase Adj. (APD 1 Gate)"() -> (w2621:i16)
        n639 = Negate(x=w2621) -> (-x=w2629:i16)
        n640 = Select(t=w2629, s="- phase (APD 1 Gate)", f=w2621) -> (s? t:f=w2628:i16)
        n641 = Or(x="- phase (APD 1 Gate)", y="+ phase (APD 1 Gate)") -> (x .or. y?=w2624:bool)
        n642 = xnode "Read/Write Control"("FPGA VI Reference In"=w2631, "error in"=w2630, "Phase count adjustment (APD 1 Gate)"=w2628) -> ("FPGA VI Reference Out"=w2626:T19, "error out"=w2627:errorcluster)
        n643 = xnode "Read/Write Control"("FPGA VI Reference In"=w2626, "error in"=w2627, "+ phase (APD 1 Gate)"=w2624) -> ("error out"=w2625:errorcluster)  [unwired: 1 out]
      }
      event "+ phase (APD 2 Gate)", "- phase (APD 2 Gate)": Value Change {
        n644 = event-data() -> ()  [unwired: 7 out]
        n645 = local read "Phase Adj. (APD 2 Gate)"() -> (w2707:i16)
        n646 = Negate(x=w2707) -> (-x=w2715:i16)
        n647 = Select(t=w2715, s="- phase (APD 2 Gate)", f=w2707) -> (s? t:f=w2714:i16)
        n648 = Or(x="- phase (APD 2 Gate)", y="+ phase (APD 2 Gate)") -> (x .or. y?=w2710:bool)
        n649 = xnode "Read/Write Control"("FPGA VI Reference In"=w2717, "error in"=w2716, "Phase count adjustment (APD 2 Gate)"=w2714) -> ("FPGA VI Reference Out"=w2712:T19, "error out"=w2713:errorcluster)
        n650 = xnode "Read/Write Control"("FPGA VI Reference In"=w2712, "error in"=w2713, "+ phase (APD 2 Gate)"=w2710) -> ("error out"=w2711:errorcluster)  [unwired: 1 out]
      }
      event "Phase Adj. (APD Acq)", "+ phase (APD Acq)", "- phase (APD Acq)": Value Change {
        n651 = event-data() -> ()  [unwired: 7 out]
        n652 = local read "Phase Adj. (APD Acq)"() -> (w2795:i16)
        n653 = Negate(x=w2795) -> (-x=w2801:i16)
        n654 = Select(t=w2801, s="+ phase (APD Acq)", f=w2795) -> (s? t:f=w2800:i16)
        n655 = Or(x="+ phase (APD Acq)", y="- phase (APD Acq)") -> (x .or. y?=w2796:bool)
        n656 = xnode "Read/Write Control"("FPGA VI Reference In"=w2803, "error in"=w2802, "Phase Count Adjustment (APD Acq)"=w2800) -> ("FPGA VI Reference Out"=w2798:T19, "error out"=w2799:errorcluster)
        n657 = xnode "Read/Write Control"("FPGA VI Reference In"=w2798, "error in"=w2799, "+ phase (APD Acq)"=w2796) -> ("error out"=w2797:errorcluster)  [unwired: 1 out]
      }
      event "Phase adj. (GI)", "+ phase (GI)", "- phase (GI)": Value Change {
        n658 = event-data() -> ()  [unwired: 7 out]
        n659 = Negate(x="Phase adj. (GI)") -> (-x=w2887:i16)
        n660 = Select(t=w2887, s="+ phase (GI)", f="Phase adj. (GI)") -> (s? t:f=w2886:i16)
        n661 = Or(x="+ phase (GI)", y="- phase (GI)") -> (x .or. y?=w2882:bool)
        n662 = xnode "Read/Write Control"("FPGA VI Reference In"=w2889, "error in"=w2888, "Phase count adjustment (GI)"=w2886) -> ("FPGA VI Reference Out"=w2884:T19, "error out"=w2885:errorcluster)
        n663 = xnode "Read/Write Control"("FPGA VI Reference In"=w2884, "error in"=w2885, "+ phase (GI)"=w2882) -> ("error out"=w2883:errorcluster)  [unwired: 1 out]
      }
      event "Phase adj. (GI) 2", "+ phase (GI) 2", "- phase (GI) 2": Value Change {
        n664 = event-data() -> ()  [unwired: 7 out]
        n665 = Negate(x="Phase adj. (GI) 2") -> (-x=w2973:i16)
        n666 = Select(t=w2973, s="+ phase (GI) 2", f="Phase adj. (GI) 2") -> (s? t:f=w2972:i16)
        n667 = Or(x="+ phase (GI) 2", y="- phase (GI) 2") -> (x .or. y?=w2968:bool)
        n668 = xnode "Read/Write Control"("FPGA VI Reference In"=w2975, "error in"=w2974, "Phase count adjustment (GI) 2"=w2972) -> ("FPGA VI Reference Out"=w2970:T19, "error out"=w2971:errorcluster)
        n669 = xnode "Read/Write Control"("FPGA VI Reference In"=w2970, "error in"=w2971, "+ phase (GI) 2"=w2968) -> ("error out"=w2969:errorcluster)  [unwired: 1 out]
      }
      event "Phase adj. (Green FB)", "- phase (Green FB)", "+ phase (Green FB)": Value Change {
        n670 = event-data() -> ()  [unwired: 7 out]
        n671 = Negate(x="Phase adj. (Green FB)") -> (-x=w3059:i16)
        n672 = Select(t=w3059, s="+ phase (Green FB)", f="Phase adj. (Green FB)") -> (s? t:f=w3058:i16)
        n673 = Or(x="+ phase (Green FB)", y="- phase (Green FB)") -> (x .or. y?=w3054:bool)
        n674 = xnode "Read/Write Control"("FPGA VI Reference In"=w3061, "error in"=w3060, "Phase count adjustment (Green FB)"=w3058) -> ("FPGA VI Reference Out"=w3056:T19, "error out"=w3057:errorcluster)
        n675 = xnode "Read/Write Control"("FPGA VI Reference In"=w3056, "error in"=w3057, "+ phase (Green FB)"=w3054) -> ("error out"=w3055:errorcluster)  [unwired: 1 out]
      }
      event "Invert APD Gate", "APD Gate ON Count", "APD Gate OFF Count", "APD Gate", "APD Integration Time (s)", "APD 1 AO Mult.", "APD 2 AO Mult.": Value Change {
        n676 = event-data() -> ()  [unwired: 7 out]
        n677 = local read "APD Integration Time (s)"() -> (w3137:dbl)
        n678 = local read "APD Gate ON Count"() -> (w3150:u32)
        n679 = local read "APD Gate OFF Count"() -> (w3149:u32)
        n680 = local read "Invert APD Gate"() -> (w3151:bool)
        n681 = local read "APD Gate"() -> (w3148:enum32{"ON", "OFF", "Interlace"})
        n682 = Multiply(x=w3137, y=40000000.0) -> (x*y=w3146:dbl)
        n683 = Reciprocal(x=w3137) -> (1/x=→"APD Acq Rate (Hz)":dbl)
        n684 = To Unsigned Long Integer(number=w3146) -> (unsigned 32bit integer=w3145:u32)
        n685 = local read "DMA Update Period (s)"() -> (w3138:dbl)
        n686 = Divide(x=w3138, y=w3137) -> (x/y=w3141:dbl)
        n687 = local read "APD 1 AO Mult."() -> (w3143:i16)
        n688 = local read "APD 2 AO Mult."() -> (w3142:i16)
        n689 = Multiply(x=2.0, y=w3141) -> (x*y=w3140:dbl)
        n690 = local write "APD Samples/FIFO Acq."(w3141) -> ()
        n691 = local write "APD Elements/DMA read"(w3140) -> ()
        n692 = xnode "Read/Write Control"("FPGA VI Reference In"=w3154, "error in"=w3153, "Invert APD Gate"=w3151, "APD Gate ON Count"=w3150, "APD Gate OFF Count"=w3149, "APD Acq Rate Count"=w3145, "APD Gate Operating Mode"=w3148, "APD 1 AO scale factor"=w3143, "APD 2 AO scale factor"=w3142) -> ("error out"=w3152:errorcluster)  [unwired: 1 out]
      }
      event "GI Frequency, ON count", "Green FB Count", "GI Frequency, OFF count": Value Change {
        n693 = event-data() -> ()  [unwired: 7 out]